vi "Dresden R2R Sputter 03.02.2018 IY24.vi"() -> ()   [LabVIEW 2009] (continued)
                                frame #0 {
                                }
                                frame #1 {
                                n27652 = local read "R_Thickness Selection"() -> (w32763:enum32{"Thickness", "Time"})
                                n27653 = case shown="\"Thickness\", Default" w32763 {
                                frame #0 {
                                n27654 = local read "Semi"() -> (w32766:bool)
                                n27655 = case shown="False" w32766 {
                                frame #0 {
                                n27656 = stacked-sequence {
                                frame #0 {
                                n27657 = local read "Semi"() -> (w32767:bool)
                                n27658 = case shown="False" w32767 {
                                frame #0 {
                                n27659 = local write "Tm2_auto_set_zero"(TRUE ("Tm1_auto_set_zero")) -> ()
                                n27660 = Wait (ms)(milliseconds to wait=u32 3000) -> ()  [unwired: 1 out]
                                }
                                frame #1 {
                                }
                                }
                                }
                                frame #1 {
                                n27661 = local read "Semi"() -> (w32770:bool)
                                n27662 = case shown="False" w32770 {
                                frame #0 {
                                n27663 = flat-sequence {
                                frame #0 {
                                n27664 = local write "Process_sputter 2"(u8 0 ("Process_sputter")) -> ()
                                }
                                frame #1 {
                                n27665 = Wait (ms)(milliseconds to wait=u32 1000) -> ()  [unwired: 1 out]
                                }
                                }
                                }
                                frame #1 {
                                }
                                }
                                }
                                frame #2 {
                                n27666 = local read "Semi"() -> (w32773:bool)
                                n27667 = case shown="False" w32773 {
                                frame #0 {
                                n27668 = local write "Process_sputter 2"(u8 0 ("Process_sputter")) -> ()
                                n27669 = property on="Process_tab_sputter 2" class="TabCtl (strict)"("Visible"=TRUE) -> ()  [unwired: 2 in, 2 out]
                                }
                                frame #1 {
                                }
                                }
                                }
                                frame #3 {
                                n27670 = local read "Semi"() -> (w32776:bool)
                                n27671 = case shown="False" w32776 {
                                frame #0 {
                                n27672 = while {
                                stop <- w32781 stop-if-true
                                n27673 = local read "R_Target Thickness Value"() -> (w32779:dbl)
                                n27674 = local read "Thickness 2-1"() -> (w32778:dbl)
                                n27675 = local read "Tm2_fail"() -> (w32789:bool)
                                n27676 = case shown="True" w32789 {
                                tunnel: [FALSE TRUE] -> w32782
                                frame #0 {
                                }
                                frame #1 {
                                n27677 = local write "Error Message"("Sputtering Process cancelled.\nPlease check TM1 connections." ("Error Message")) -> ()
                                }
                                }
                                n27678 = Divide(x=w32778, y=w32779) -> (x/y=w32787:dbl)
                                n27679 = Multiply(x=w32787, y=100.0) -> (x*y=w32785:dbl)
                                n27680 = Greater Or Equal?(x=w32785, y=100.0) -> (x >= y?=w32784:bool)
                                n27681 = local write "Target Thickness Sputter 2"(w32779) -> ()
                                n27682 = local write "Thickness_total 2"(w32778) -> ()
                                n27683 = local read "Abort_sputter 2"() -> (w32777:bool)
                                n27684 = local write "Process_sputter 2"(w32785) -> ()
                                n27685 = Wait Until Next ms Multiple(millisecond multiple=u32 300) -> ()  [unwired: 1 out]
                                n27686 = local read "Semi"() -> (w32783:bool)
                                n27687 = Compound Arithmetic op=OR(w32783, w32784, w32777, w32782) -> (w32781:bool)
                                }
                                }
                                frame #1 {
                                }
                                }
                                }
                                frame #4 {
                                n27688 = local read "Semi"() -> (w32793:bool)
                                n27689 = case shown="False" w32793 {
                                frame #0 {
                                w32794 = FALSE ("Abort_sputter")
                                n27690 = local write "Abort_sputter 2"(w32794) -> ()
                                n27691 = property on="Process_tab_sputter 2" class="TabCtl (strict)"("Visible"=w32794) -> ()  [unwired: 2 in, 2 out]
                                }
                                frame #1 {
                                }
                                }
                                }
                                frame #5 {
                                n27692 = local read "Tm1_fail"() -> (w32795:bool)
                                n27693 = case shown="False" w32795 {
                                frame #0 {
                                n27694 = Wait (ms)(milliseconds to wait=u32 1000) -> ()  [unwired: 1 out]
                                n27695 = local write "SDC1 23"(TRUE ("SDC1 23")) -> ()
                                }
                                frame #1 {
                                }
                                }
                                }
                                }
                                }
                                frame #1 {
                                }
                                }
                                }
                                frame #1 {
                                n27696 = local read "Semi"() -> (w32798:bool)
                                n27697 = case shown="False" w32798 {
                                frame #0 {
                                n27698 = stacked-sequence {
                                frame #0 {
                                n27699 = local read "Semi"() -> (w32799:bool)
                                n27700 = case shown="False" w32799 {
                                frame #0 {
                                w32800 = TRUE ("Tm1_auto_set_zero")
                                n27701 = local write "Tm2_auto_set_zero"(w32800) -> ()
                                n27702 = property on="Sputter_tab 2" class="TabCtl (strict)"("Visible"=w32800) -> ()  [unwired: 2 in, 2 out]
                                n27703 = Wait (ms)(milliseconds to wait=u32 1000) -> ()  [unwired: 1 out]
                                }
                                frame #1 {
                                }
                                }
                                }
                                frame #1 {
                                n27704 = local read "Semi"() -> (w32802:bool)
                                n27705 = case shown="False" w32802 {
                                frame #0 {
                                n27706 = while {
                                i -> [w32811]
                                stop <- w32810 stop-if-true
                                n27707 = Wait Until Next ms Multiple(millisecond multiple=u32 1000) -> ()  [unwired: 1 out]
                                n27708 = local read "R_Duration"() -> (w32812:dbl)
                                n27709 = local read "Sputter_cancel 2"() -> (w32803:bool)
                                n27710 = local read "Semi"() -> (w32807:bool)
                                n27711 = Multiply(x=w32812, y=60.0) -> (x*y=w32809:dbl)
                                n27712 = Greater?(x=w32811, y=w32809) -> (0:w32808:bool)
                                n27713 = Compound Arithmetic op=OR(w32807, w32803, w32808) -> (w32806:bool)
                                n27714 = local read "R_Duration"() -> (w32804:dbl)
                                n27715 = case shown="True" w32806 {
                                tunnel: w32811 -> [w32816 _]
                                tunnel: [FALSE TRUE] -> w32810
                                tunnel: w32809 -> [w32817 _]
                                frame #0 {
                                n27716 = Subtract(x=w32817, y=w32816) -> (x-y=w32814:dbl)
                                n27717 = local write "Sputter_left_time 2"(w32814) -> ()
                                }
                                frame #1 {
                                n27718 = property on="Sputter_tab 2" class="TabCtl (strict)"("Visible"=FALSE) -> ()  [unwired: 2 in, 2 out]
                                }
                                }
                                n27719 = local write "Sputter_set_time 2"(w32804) -> ()
                                }
                                }
                                frame #1 {
                                }
                                }
                                }
                                frame #2 {
                                n27720 = local write "Sputter_cancel 2"(FALSE ("Sputter_cancel")) -> ()
                                }
                                frame #3 {
                                n27721 = local write "SDC1 24"(TRUE ("SDC1 24")) -> ()
                                n27722 = Wait (ms)(milliseconds to wait=u32 1000) -> ()  [unwired: 1 out]
                                }
                                }
                                }
                                frame #1 {
                                }
                                }
                                }
                                }
                                n27723 = local read "Substrate Material"() -> (w32764:string)
                                n27724 = Write to Text File(file (use dialog)=path path "D/VK-1701 System Files/Material Data/data2.txt", text=w32764) -> ()  [unwired: 2 in, 3 out]
                                }
                                }
                                }
                                frame #1 {
                                }
                                }
                                }
                                frame #20 {
                                # "CLOSE DC"
                                n27725 = local read "Semi"() -> (w32823:bool)
                                n27726 = case shown="False" w32823 {
                                frame #0 {
                                n27727 = stacked-sequence {
                                frame #0 {
                                n27728 = local read "Semi"() -> (w32824:bool)
                                n27729 = case shown="False" w32824 {
                                frame #0 {
                                n27730 = local write "Dc_auto_off"(TRUE ("Dc_auto_off")) -> ()
                                }
                                frame #1 {
                                }
                                }
                                }
                                frame #1 {
                                n27731 = local read "Semi"() -> (w32826:bool)
                                n27732 = case shown="False" w32826 {
                                frame #0 {
                                n27733 = Wait (ms)(milliseconds to wait=u32 1000) -> ()  [unwired: 1 out]
                                }
                                frame #1 {
                                }
                                }
                                }
                                frame #2 {
                                n27734 = local read "Semi"() -> (w32828:bool)
                                n27735 = case shown="False" w32828 {
                                frame #0 {
                                n27736 = local write "Dc_auto_set_zero"(TRUE ("Dc_auto_set")) -> ()
                                }
                                frame #1 {
                                }
                                }
                                }
                                frame #3 {
                                n27737 = local read "Semi"() -> (w32830:bool)
                                n27738 = case shown="False" w32830 {
                                frame #0 {
                                n27739 = Wait (ms)(milliseconds to wait=u32 1000) -> ()  [unwired: 1 out]
                                }
                                frame #1 {
                                }
                                }
                                }
                                frame #4 {
                                n27740 = local read "Semi"() -> (w32832:bool)
                                n27741 = case shown="False" w32832 {
                                frame #0 {
                                n27742 = while {
                                i -> [w32844]
                                stop <- w32833 stop-if-true
                                n27743 = Greater?(x=w32844, y=600) -> (0:w32843:bool)
                                n27744 = case shown="True" w32843 {
                                frame #0 {
                                }
                                frame #1 {
                                n27745 = local write "Semi"(TRUE ("Semi")) -> ()
                                n27746 = local write "Error Message"("Sputter Process cancelled.\nPlease Check DC connections." ("Error Message")) -> ()
                                }
                                }
                                n27747 = local read "Actual DC Power : 2"() -> (w32838:dbl)
                                n27748 = local read "Actual DC Volt2"() -> (w32837:dbl)
                                n27749 = Less?(x=w32838, y=10.0) -> (x < y?=w32841:bool)
                                n27750 = Less?(x=w32837, y=20.0) -> (x < y?=w32842:bool)
                                n27751 = And(x=w32841, y=w32842) -> (x .and. y?=w32835:bool)
                                n27752 = local read "Semi"() -> (w32834:bool)
                                n27753 = Wait Until Next ms Multiple(millisecond multiple=u32 500) -> ()  [unwired: 1 out]
                                n27754 = Compound Arithmetic op=OR(w32835, w32834) -> (w32833:bool)
                                }
                                }
                                frame #1 {
                                }
                                }
                                }
                                frame #5 {
                                n27755 = local read "Semi"() -> (w32848:bool)
                                n27756 = case shown="False" w32848 {
                                frame #0 {
                                n27757 = while {
                                i -> [w32854]
                                stop <- w32849 stop-if-true
                                n27758 = Greater?(x=w32854, y=50) -> (0:w32853:bool)
                                n27759 = case shown="True" w32853 {
                                frame #0 {
                                }
                                frame #1 {
                                n27760 = local write "Semi"(TRUE ("Semi")) -> ()
                                n27761 = local write "Error Message"("Sputter Process cancelled.\nPlease Check DCPS-SW2." ("Error Message")) -> ()
                                }
                                }
                                n27762 = local read "Cnt_Dcps_sw2_di"() -> (w32852:bool)
                                n27763 = case shown="True" w32852 {
                                tunnel: [TRUE ("Cnt_Dcps_sw1_do") FALSE ("Cnt_Dcps_sw1_do")] -> w32851
                                frame #0 {
                                }
                                frame #1 {
                                n27764 = local write "Cnt_Dcps_sw2_do"(FALSE ("Cnt_Dcps_sw1_do")) -> ()
                                n27765 = Wait Until Next ms Multiple(millisecond multiple=u32 500) -> ()  [unwired: 1 out]
                                }
                                }
                                n27766 = local read "Semi"() -> (w32850:bool)
                                n27767 = Or(x=w32851, y=w32850) -> (x .or. y?=w32849:bool)
                                }
                                }
                                frame #1 {
                                }
                                }
                                }
                                frame #6 {
                                n27768 = local read "Semi"() -> (w32862:bool)
                                n27769 = case shown="False" w32862 {
                                frame #0 {
                                n27770 = Wait (ms)(milliseconds to wait=u32 1000) -> ()  [unwired: 1 out]
                                n27771 = local write "SDC1 25"(TRUE ("SDC1 25")) -> ()
                                }
                                frame #1 {
                                }
                                }
                                }
                                }
                                }
                                frame #1 {
                                }
                                }
                                }
                                frame #21 {
                                # "PC-BV OPEN"
                                n27772 = stacked-sequence {
                                frame #0 {
                                n27773 = local read "Semi"() -> (w32865:bool)
                                n27774 = case shown="False" w32865 {
                                frame #0 {
                                n27775 = stacked-sequence {
                                frame #0 {
                                n27776 = local read "Semi"() -> (w32866:bool)
                                n27777 = case shown="False" w32866 {
                                frame #0 {
                                n27778 = local write "Pc_bv3_auto_open"(TRUE ("Tp1_auto_start")) -> ()
                                }
                                frame #1 {
                                }
                                }
                                }
                                frame #1 {
                                n27779 = local read "Semi"() -> (w32868:bool)
                                n27780 = case shown="False" w32868 {
                                frame #0 {
                                n27781 = Wait (ms)(milliseconds to wait=u32 1000) -> ()  [unwired: 1 out]
                                }
                                frame #1 {
                                }
                                }
                                }
                                frame #2 {
                                n27782 = local read "Semi"() -> (w32870:bool)
                                n27783 = case shown="False" w32870 {
                                frame #0 {
                                n27784 = while {
                                i -> [w32876]
                                stop <- w32872 stop-if-true
                                n27785 = local read "Pc_bv_opened_ch3"() -> (w32874:bool)
                                n27786 = Greater?(x=w32876, y=120) -> (0:w32875:bool)
                                n27787 = local read "Semi"() -> (w32873:bool)
                                n27788 = Compound Arithmetic op=OR(w32873, w32874, w32875) -> (w32872:bool)
                                n27789 = Wait (ms)(milliseconds to wait=u32 500) -> ()  [unwired: 1 out]
                                }
                                }
                                frame #1 {
                                }
                                }
                                }
                                frame #3 {
                                n27790 = local read "Semi"() -> (w32878:bool)
                                n27791 = case shown="False" w32878 {
                                frame #0 {
                                n27792 = local read "Pc_bv_opened_ch3"() -> (w32879:bool)
                                n27793 = case shown="False" w32879 {
                                frame #0 {
                                n27794 = local write "Pc_bv3_auto_open"(TRUE ("Pc_bv1_auto_open")) -> ()
                                }
                                frame #1 {
                                }
                                }
                                }
                                frame #1 {
                                }
                                }
                                }
                                frame #4 {
                                n27795 = local read "Semi"() -> (w32881:bool)
                                n27796 = case shown="False" w32881 {
                                frame #0 {
                                n27797 = local read "Pc_bv_opened_ch3"() -> (w32882:bool)
                                n27798 = case shown="False" w32882 {
                                frame #0 {
                                n27799 = Wait (ms)(milliseconds to wait=u32 1000) -> ()  [unwired: 1 out]
                                }
                                frame #1 {
                                }
                                }
                                }
                                frame #1 {
                                }
                                }
                                }
                                frame #5 {
                                n27800 = local read "Semi"() -> (w32884:bool)
                                n27801 = case shown="False" w32884 {
                                frame #0 {
                                n27802 = while {
                                i -> [w32890]
                                stop <- w32886 stop-if-true
                                n27803 = local read "Pc_bv_opened_ch3"() -> (w32888:bool)
                                n27804 = Greater?(x=w32890, y=120) -> (0:w32889:bool)
                                n27805 = local read "Semi"() -> (w32887:bool)
                                n27806 = Compound Arithmetic op=OR(w32887, w32888, w32889) -> (w32886:bool)
                                n27807 = Wait (ms)(milliseconds to wait=u32 500) -> ()  [unwired: 1 out]
                                }
                                }
                                frame #1 {
                                }
                                }
                                }
                                frame #6 {
                                n27808 = local read "Semi"() -> (w32892:bool)
                                n27809 = case shown="False" w32892 {
                                frame #0 {
                                n27810 = local read "Pc_bv_opened_ch3"() -> (w32893:bool)
                                n27811 = case shown="False" w32893 {
                                frame #0 {
                                n27812 = local write "Error Message"("Start up process  cancelled\nbecause  PC-BV not opened.\nPlease check PC-BV1 connections." ("Error Message")) -> ()
                                n27813 = Wait (ms)(milliseconds to wait=u32 1000) -> ()  [unwired: 1 out]
                                }
                                frame #1 {
                                }
                                }
                                }
                                frame #1 {
                                }
                                }
                                }
                                }
                                }
                                frame #1 {
                                }
                                }
                                }
                                frame #1 {
                                n27814 = local read "Semi"() -> (w32896:bool)
                                n27815 = case shown="False" w32896 {
                                frame #0 {
                                n27816 = Wait (ms)(milliseconds to wait=u32 1000) -> ()  [unwired: 1 out]
                                n27817 = local write "SDC1 28"(TRUE ("SDC1 28")) -> ()
                                }
                                frame #1 {
                                }
                                }
                                }
                                }
                                }
                                frame #22 {
                                # "set ar zero"
                                n27818 = stacked-sequence {
                                frame #0 {
                                n27819 = local read "Semi"() -> (w32899:bool)
                                n27820 = case shown="False" w32899 {
                                frame #0 {
                                n27821 = stacked-sequence {
                                frame #0 {
                                n27822 = local read "Semi"() -> (w32900:bool)
                                n27823 = case shown="False" w32900 {
                                frame #0 {
                                n27824 = local write "Ar_auto_set_zero_ch3"(TRUE ("Ar_auto_set_zero_ch1")) -> ()
                                }
                                frame #1 {
                                }
                                }
                                }
                                frame #1 {
                                n27825 = local read "Semi"() -> (w32902:bool)
                                n27826 = case shown="False" w32902 {
                                frame #0 {
                                n27827 = while {
                                i -> [w32905]
                                stop <- w32904 stop-if-true
                                n27828 = Greater?(x=w32905, y=150) -> (0:w32904:bool)
                                n27829 = local read "Semi"() -> (w32903:bool)
                                n27830 = case shown="False" w32903 {
                                tunnel: [FALSE TRUE] -> _
                                frame #0 {
                                n27831 = Wait Until Next ms Multiple(millisecond multiple=u32 200) -> ()  [unwired: 1 out]
                                }
                                frame #1 {
                                }
                                }
                                }
                                }
                                frame #1 {
                                }
                                }
                                }
                                frame #2 {
                                n27832 = local read "Semi"() -> (w32910:bool)
                                n27833 = case shown="False" w32910 {
                                frame #0 {
                                n27834 = local read "Ar_sccm_act 2"() -> (w32911:dbl)
                                n27835 = Less?(x=w32911, y=1) -> (x < y?=w32912:bool)
                                n27836 = case shown="False" w32912 {
                                frame #0 {
                                n27837 = local write "Ar_auto_set_zero_ch3"(TRUE ("Ar_auto_set_zero_ch1")) -> ()
                                }
                                frame #1 {
                                }
                                }
                                }
                                frame #1 {
                                }
                                }
                                }
                                frame #3 {
                                n27838 = local read "Semi"() -> (w32915:bool)
                                n27839 = case shown="False" w32915 {
                                frame #0 {
                                n27840 = local read "Ar_sccm_act 2"() -> (w32916:dbl)
                                n27841 = Less?(x=w32916, y=1) -> (x < y?=w32917:bool)
                                n27842 = case shown="False" w32917 {
                                frame #0 {
                                n27843 = while {
                                i -> [w32923]
                                stop <- w32920 stop-if-true
                                n27844 = Greater?(x=w32923, y=150) -> (0:w32921:bool)
                                n27845 = local read "Semi"() -> (w32919:bool)
                                n27846 = case shown="True" w32919 {
                                tunnel: [FALSE FALSE] -> w32922
                                frame #0 {
                                }
                                frame #1 {
                                n27847 = Wait Until Next ms Multiple(millisecond multiple=u32 200) -> ()  [unwired: 1 out]
                                }
                                }
                                n27848 = Or(x=w32922, y=w32921) -> (x .or. y?=w32920:bool)
                                }
                                }
                                frame #1 {
                                }
                                }
                                }
                                frame #1 {
                                }
                                }
                                }
                                frame #4 {
                                n27849 = local read "Semi"() -> (w32928:bool)
                                n27850 = case shown="False" w32928 {
                                frame #0 {
                                n27851 = Wait (ms)(milliseconds to wait=u32 1000) -> ()  [unwired: 1 out]
                                }
                                frame #1 {
                                }
                                }
                                }
                                }
                                }
                                frame #1 {
                                }
                                }
                                }
                                frame #1 {
                                n27852 = local read "Semi"() -> (w32930:bool)
                                n27853 = case shown="False" w32930 {
                                frame #0 {
                                n27854 = local write "SDC1 26"(TRUE ("SDC1 26")) -> ()
                                n27855 = Wait (ms)(milliseconds to wait=u32 1000) -> ()  [unwired: 1 out]
                                }
                                frame #1 {
                                }
                                }
                                }
                                }
                                }
                                frame #23 {
                                # "sov-ar close"
                                n27856 = stacked-sequence {
                                frame #0 {
                                n27857 = local read "Semi"() -> (w32933:bool)
                                n27858 = case shown="False" w32933 {
                                frame #0 {
                                n27859 = while {
                                i -> [w32939]
                                stop <- w32934 stop-if-true
                                n27860 = Greater?(x=w32939, y=50) -> (0:w32938:bool)
                                n27861 = case shown="True" w32938 {
                                frame #0 {
                                }
                                frame #1 {
                                n27862 = local write "Semi"(TRUE ("Semi")) -> ()
                                n27863 = local write "Error Message"("Coating Process  \nwas cancelled.\nPlease check \nSOV-Ar connection." ("Error Message")) -> ()
                                }
                                }
                                n27864 = local read "Ch3_Sov_Ar_di"() -> (w32937:bool)
                                n27865 = case shown="True" w32937 {
                                tunnel: [TRUE FALSE] -> w32936
                                frame #0 {
                                }
                                frame #1 {
                                n27866 = local write "Ch3_Sov_Ar_do"(FALSE ("Ch1_WFC_do")) -> ()
                                n27867 = Wait Until Next ms Multiple(millisecond multiple=u32 200) -> ()  [unwired: 1 out]
                                }
                                }
                                n27868 = local read "Semi"() -> (w32935:bool)
                                n27869 = Or(x=w32936, y=w32935) -> (x .or. y?=w32934:bool)
                                }
                                }
                                frame #1 {
                                }
                                }
                                }
                                frame #1 {
                                n27870 = local read "Semi"() -> (w32947:bool)
                                n27871 = case shown="False" w32947 {
                                frame #0 {
                                n27872 = local write "SDC1 27"(TRUE ("SDC1 27")) -> ()
                                n27873 = Wait (ms)(milliseconds to wait=u32 1000) -> ()  [unwired: 1 out]
                                }
                                frame #1 {
                                }
                                }
                                }
                                }
                                }
                                frame #24 {
                                # "CC OPEN"
                                n27874 = stacked-sequence {
                                frame #0 {
                                n27875 = local read "Semi"() -> (w32950:bool)
                                n27876 = case shown="False" w32950 {
                                frame #0 {
                                n27877 = while {
                                i -> [w32956]
                                stop <- w32951 stop-if-true
                                n27878 = Greater?(x=w32956, y=50) -> (0:w32955:bool)
                                n27879 = case shown="True" w32955 {
                                frame #0 {
                                }
                                frame #1 {
                                n27880 = local write "Semi"(TRUE ("Semi")) -> ()
                                n27881 = local write "Error Message"("Coating Process  \nwas cancelled.\nPlease check \nBG-BV connection." ("Error Message")) -> ()
                                }
                                }
                                n27882 = local read "Ch3_Cc_on_off_di"() -> (w32954:bool)
                                n27883 = case shown="False" w32954 {
                                tunnel: [FALSE TRUE] -> w32953
                                frame #0 {
                                n27884 = local write "Ch3_Cc_on_off_do"(TRUE ("Ch1_WFC_do")) -> ()
                                n27885 = Wait Until Next ms Multiple(millisecond multiple=u32 200) -> ()  [unwired: 1 out]
                                }
                                frame #1 {
                                }
                                }
                                n27886 = local read "Semi"() -> (w32952:bool)
                                n27887 = Or(x=w32953, y=w32952) -> (x .or. y?=w32951:bool)
                                }
                                }
                                frame #1 {
                                }
                                }
                                }
                                frame #1 {
                                n27888 = local read "Semi"() -> (w32964:bool)
                                n27889 = case shown="False" w32964 {
                                frame #0 {
                                n27890 = while {
                                i -> [w32969]
                                stop <- w32967 stop-if-true
                                n27891 = Greater?(x=w32969, y=30) -> (0:w32965:bool)
                                n27892 = Wait Until Next ms Multiple(millisecond multiple=u32 1000) -> ()  [unwired: 1 out]
                                n27893 = local read "Semi"() -> (w32968:bool)
                                n27894 = Or(x=w32965, y=w32968) -> (x .or. y?=w32967:bool)
                                }
                                }
                                frame #1 {
                                }
                                }
                                }
                                frame #2 {
                                n27895 = local read "Semi"() -> (w32971:bool)
                                n27896 = case shown="False" w32971 {
                                frame #0 {
                                n27897 = local write "SDC1 27b"(TRUE ("SDC1 3")) -> ()
                                n27898 = Wait (ms)(milliseconds to wait=u32 1000) -> ()  [unwired: 1 out]
                                }
                                frame #1 {
                                }
                                }
                                }
                                }
                                }
                                frame #25 {
                                # "CHECK CHAMBER PRESSURE"
                                n27899 = stacked-sequence {
                                frame #0 {
                                n27900 = local read "Semi"() -> (w32974:bool)
                                n27901 = case shown="False" w32974 {
                                frame #0 {
                                n27902 = while {
                                i -> [w32982]
                                stop <- w32976 stop-if-true
                                n27903 = Greater?(x=w32982, y=300) -> (0:w32981:bool)
                                n27904 = case shown="True" w32981 {
                                frame #0 {
                                }
                                frame #1 {
                                n27905 = local write "Semi"(TRUE ("Semi")) -> ()
                                n27906 = local write "Error Message"("Coating Process cancelled.\nPlease check chamber \nconnections." ("Error Message")) -> ()
                                }
                                }
                                n27907 = local read "Ch_CC_press_ch3 2"() -> (w32975:dbl)
                                n27908 = Greater Or Equal?(x=w32975, y=5e-05 ("CHAMBER PRESSURE 6")) -> (x >= y?=w32979:bool)
                                n27909 = case shown="True" w32979 {
                                tunnel: [TRUE FALSE] -> w32978
                                frame #0 {
                                }
                                frame #1 {
                                n27910 = Wait Until Next ms Multiple(millisecond multiple=u32 200) -> ()  [unwired: 1 out]
                                }
                                }
                                n27911 = local read "Semi"() -> (w32977:bool)
                                n27912 = Or(x=w32978, y=w32977) -> (x .or. y?=w32976:bool)
                                }
                                }
                                frame #1 {
                                }
                                }
                                }
                                frame #1 {
                                n27913 = local read "Semi"() -> (w32989:bool)
                                n27914 = case shown="False" w32989 {
                                frame #0 {
                                n27915 = Wait (ms)(milliseconds to wait=u32 1000) -> ()  [unwired: 1 out]
                                n27916 = local write "SDC1 27c"(TRUE ("SDC1 10")) -> ()
                                }
                                frame #1 {
                                }
                                }
                                }
                                }
                                }
                                frame #26 {
                                # "encoder info  add to other web selection"
                                n27917 = stacked-sequence {
                                frame #0 {
                                n27918 = local read "Semi"() -> (w32992:bool)
                                n27919 = case shown="False" w32992 {
                                frame #0 {
                                n27920 = local read "R_Web_selection"() -> (w32993:enum32{"Web", "Other"})
                                n27921 = case shown="\"Web\", Default" w32993 {
                                frame #0 {
                                # "TC -ROLL"
                                n27922 = local read "Semi"() -> (w32994:bool)
                                n27923 = case shown="False" w32994 {
                                frame #0 {
                                n27924 = stacked-sequence {
                                frame #0 {
                                n27925 = local read "R Maximum diameter"() -> (w32996:dbl)
                                n27926 = local write "Change_Max Diameter"(w32996) -> ()
                                n27927 = Wait (ms)(milliseconds to wait=u32 300) -> ()  [unwired: 1 out]
                                }
                                frame #1 {
                                n27928 = local read "R Single DC Step1 Coating Power Active"() -> (w32997:bool)
                                n27929 = local read "R Single DC Step2 Coating Power Active"() -> (w32998:bool)
                                n27930 = local read "R Single DC Step3 Coating Power Active"() -> (w32999:bool)
                                n27931 = local read "R Single DC Step4 Coating Power Active"() -> (w33000:bool)
                                n27932 = local read "R Single DC Step5 Coating Power Active"() -> (w33001:bool)
                                n27933 = Boolean To (0,1)(Boolean=w32997) -> (0, 1=w33002:i16)
                                n27934 = Boolean To (0,1)(Boolean=w32998) -> (0, 1=w33003:i16)
                                n27935 = Boolean To (0,1)(Boolean=w32999) -> (0, 1=w33004:i16)
                                n27936 = Boolean To (0,1)(Boolean=w33000) -> (0, 1=w33005:i16)
                                n27937 = Boolean To (0,1)(Boolean=w33001) -> (0, 1=w33006:i16)
                                n27938 = Compound Arithmetic op=ADD(w33002, w33003, w33004, w33005, w33006) -> (w33008:i16)
                                n27939 = local read "R Single DC Interval length"() -> (w33007:dbl)
                                n27940 = Multiply(x=w33007, y=w33008) -> (x*y=w33009:dbl)
                                n27941 = local write "Total length"(w33009) -> ()
                                }
                                frame #2 {
                                n27942 = local write "Calculate 3"(TRUE ("Calculate_auto")) -> ()
                                }
                                frame #3 {
                                n27943 = Wait (ms)(milliseconds to wait=u32 1000) -> ()  [unwired: 1 out]
                                }
                                frame #4 {
                                n27944 = local read "Change_Max Diameter"() -> (w33013:dbl)
                                n27945 = Wait (ms)(milliseconds to wait=u32 200) -> ()  [unwired: 1 out]
                                n27946 = local write "Initial Min Diameter"(w33013) -> ()
                                }
                                frame #5 {
                                n27947 = local write "Calculate 2"(TRUE ("Calculate_auto")) -> ()
                                }
                                frame #6 {
                                n27948 = local write "Roll_side_select"(enum32{"Left to Right", "Right to Left"}."Right to Left" ("Roll_side_select")) -> ()